vi "2_VisualizeModulePositioning2_Nolan.vi"(0 "Placement Monitor":T1(plugin-control)=refnum, 1 "Calibrated positions of fiducials [mm]":dbl[][](array[numeric])=[[-658.867386146, 115.937184375, -18.342965965], [-563.38738772, 115.95451918, -18.342965965], [-563.369748267, 18.796520782, -18.342965965], [-658.849746693, 18.779185977, -18.342965965], [-560.867387761, 115.954976697, -18.342965965], [-465.387389335, 115.972311502, -18.342965965], [-465.369749882, 18.814313103, -18.342965965], [-560.849748308, 18.796978298, -18.342965965], [-462.867389377, 115.972769019, -18.342965965], [-367.38739095, 115.990103824, -18.342965965], [-367.369751497, 18.832105425, -18.342965965], [-462.849749923, 18.81477062, -18.342965965], [-364.867390992, 115.990561341, -18.342965965], [-269.387392565, 116.007896146, -18.342965965], [-269.369753112, 18.849897747, -18.342965965], [-364.849751539, 18.832562942, -18.342965965], [-266.867392607, 116.008353663, -18.342965965], [-171.38739418, 116.025688468, -18.342965965], [-171.369754727, 18.867690069, -18.342965965], [-266.849753154, 18.850355264, -18.342965965], [-168.867394222, 116.026145985, -18.342965965], [-73.387395796, 116.04348079, -18.342965965], [-73.369756342, 18.885482391, -18.342965965], [-168.849754769, 18.868147586, -18.342965965], [-70.867395837, 116.043938306, -18.342965965], [24.612602589, 116.061273111, -18.342965965], [24.630242042, 18.903274713, -18.342965965], [-70.849756384, 18.885939908, -18.342965965], [27.132602548, 116.061730628, -18.342965965], [122.612600974, 116.079065433, -18.342965965], [122.630240427, 18.921067035, -18.342965965], [27.150242001, 18.90373223, -18.342965965], [125.132600933, 116.07952295, -18.342965965], [220.612599359, 116.096857755, -18.342965965], [220.630238812, 18.938859356, -18.342965965], [125.150240386, 18.921524551, -18.342965965], [223.132599318, 116.097315272, -18.342965965], [318.612597744, 116.114650077, -18.342965965], [318.630237197, 18.956651678, -18.342965965], [223.150238771, 18.939316873, -18.342965965], [321.132597702, 116.115107594, -18.342965965], [416.612596129, 116.132442399, -18.342965965], [416.630235582, 18.974444, -18.342965965], [321.150237156, 18.957109195, -18.342965965], [419.132596087, 116.132899916, -18.342965965], [514.612594514, 116.150234721, -18.342965965], [514.630233967, 18.992236322, -18.342965965], [419.15023554, 18.974901517, -18.342965965], [517.132594472, 116.150692238, -18.342965965], [612.612592899, 116.168027043, -18.342965965], [612.630232352, 19.010028644, -18.342965965], [517.150233925, 18.992693839, -18.342965965]], 2 "XYZ .NET Refnum in":refnum<k24>, 3 "Axis Speeds":T10={"X [mm/s]"=25.0, "Y [mm/s]"=25.0, "Z [mm/s]"=25.0}, 4 "Module fiducial marker":T7=enum."Mark C", 5 "N modules":i32=13, 6 "Sensor Pattern":T8(ring)=enum."ATLAS12", 7 "error in (no error)":errorcluster, 8 "Templates path":path=path "C:/Users/Aerotech/Documents/BNL_ThermomechanicalStave", 9 "Calibration [um/pix]":dbl=1.55, 10 "Current Build Phase":refnum<vi>, 11 "Temperature":refnum<vi>, 12 "Module #":refnum<vi>, 13 "Placement tolerance [um]":dbl=25.0, 14 "Tape Type":T5=enum."Axial (Sutcliffe NP49-01-100 01-Mar-16)", 16 "Module Report":refnum<vi>, 17 "Base notes":string, 18 "Reports path":path=path "C:/Users/Aerotech/cernbox/BNL/Stave Assembly Records/2017-05-15/ModulePlacement") -> (19 "Recalibrated??":bool, 22 "XYZ .NET Refnum out":refnum<k24>, 27 "error out":errorcluster)   [LabVIEW 2016] (continued)
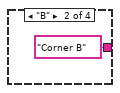
[diagram p4: hidden frame]
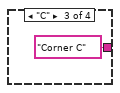
[diagram p5: hidden frame]
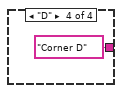
[diagram p6: hidden frame]
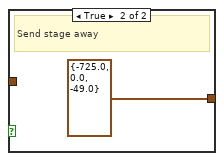
[diagram p7: hidden frame]
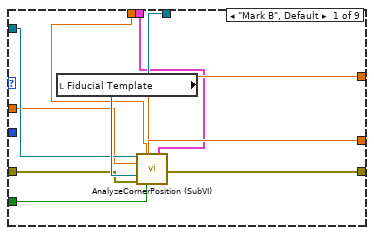
[diagram p8: hidden frame]
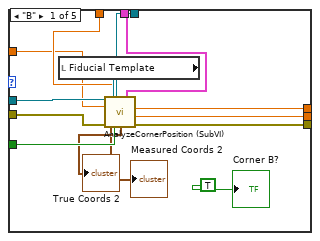
[diagram p9: hidden frame]
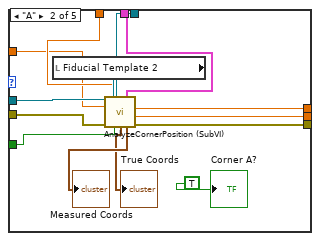
[diagram p10: hidden frame]
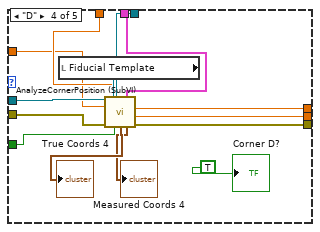
[diagram p11: hidden frame]
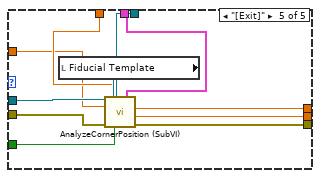
[diagram p12: hidden frame]
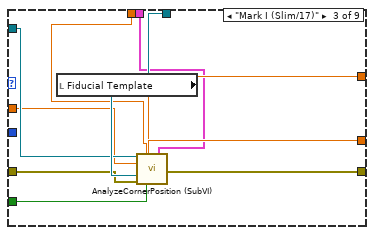
[diagram p13: hidden frame]
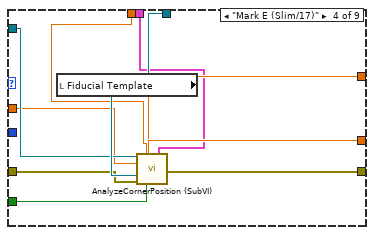
[diagram p14: hidden frame]
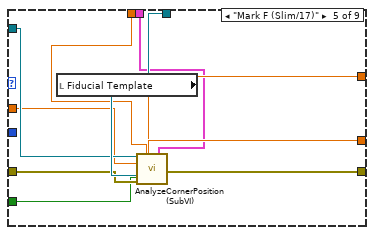
[diagram p15: hidden frame]
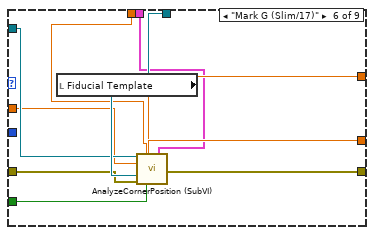
[diagram p16: hidden frame]
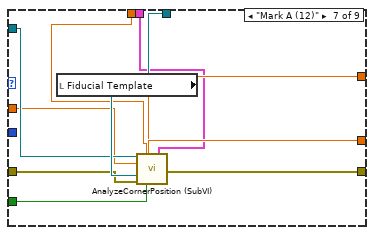
[diagram p17: hidden frame]
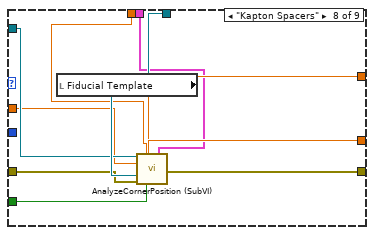
[diagram p18: hidden frame]
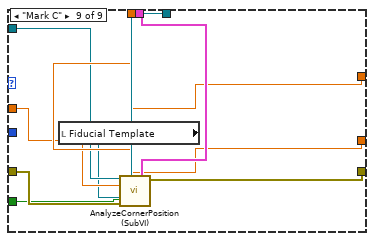
[diagram p19: hidden frame]
                                "Corner B?" <- TRUE
                              }
                              frame "A" {
                                n57 = local read "Fiducial Template 2"() -> (w249:T1)
                                n58 = call "AnalyzeCornerPosition (SubVI).vi"("Refnum in"=w244, "Placement tolerance [um]"=w242, "Calibration [um/pix]"=w240, "Fiducial Template"=w249, "error in (no error)"=w248, "Center-only search?"=w239) -> ("Offset interpreter"=w241:T3, "Refnum out"=w243:T1, "X offset [um]"=w245:sgl, "Y offset [um]"=w246:sgl, "True Coords"=→"True Coords":cluster{"X coordinate":dbl, "Y coordinate":dbl}, "Measured Coords"=→"Measured Coords":cluster{"x":sgl, "y":sgl}, "error out"=w247:errorcluster)  [unwired: 3 in]
                                "Corner A?" <- TRUE
                              }
                              frame "C" {
                                n59 = local read "Fiducial Template 2"() -> (w263:T1)
                                n60 = call "AnalyzeCornerPosition (SubVI).vi"("Refnum in"=w258, "Placement tolerance [um]"=w256, "Calibration [um/pix]"=w254, "Fiducial Template"=w263, "error in (no error)"=w262, "Center-only search?"=w253) -> ("Offset interpreter"=w255:T3, "Refnum out"=w257:T1, "X offset [um]"=w259:sgl, "Y offset [um]"=w260:sgl, "True Coords"=→"True Coords 3":cluster{"X coordinate":dbl, "Y coordinate":dbl}, "Measured Coords"=→"Measured Coords 3":cluster{"x":sgl, "y":sgl}, "error out"=w261:errorcluster)  [unwired: 3 in]
                                "Corner C?" <- TRUE
                              }
                              frame "D" {
                                n61 = local read "Fiducial Template"() -> (w277:T1)
                                n62 = call "AnalyzeCornerPosition (SubVI).vi"("Refnum in"=w272, "Placement tolerance [um]"=w270, "Calibration [um/pix]"=w268, "Fiducial Template"=w277, "error in (no error)"=w276, "Center-only search?"=w267) -> ("Offset interpreter"=w269:T3, "Refnum out"=w271:T1, "X offset [um]"=w273:sgl, "Y offset [um]"=w274:sgl, "True Coords"=→"True Coords 4":cluster{"X coordinate":dbl, "Y coordinate":dbl}, "Measured Coords"=→"Measured Coords 4":cluster{"x":sgl, "y":sgl}, "error out"=w275:errorcluster)  [unwired: 3 in]
                                "Corner D?" <- TRUE
                              }
                              frame "[Exit]" {
                                n63 = local read "Fiducial Template"() -> (w288:T1)
                                n64 = call "AnalyzeCornerPosition (SubVI).vi"("Refnum in"=w283, "Placement tolerance [um]"=w281, "Calibration [um/pix]"=w279, "Fiducial Template"=w288, "error in (no error)"=w287, "Center-only search?"=w278) -> ("Offset interpreter"=w280:T3, "Refnum out"=w282:T1, "X offset [um]"=w284:sgl, "Y offset [um]"=w285:sgl, "error out"=w286:errorcluster)  [unwired: 3 in, 2 out]
                              }
                            }
                          }
                          frame "Mark I (Slim/17)" {
                            n65 = local read "Fiducial Template"() -> (w299:T1)
                            n66 = call "AnalyzeCornerPosition (SubVI).vi"("Refnum in"=w294, "Placement tolerance [um]"=w292, "Calibration [um/pix]"=w290, "Fiducial Template"=w299, "error in (no error)"=w298, "Center-only search?"=w289) -> ("Offset interpreter"=w291:T3, "Refnum out"=w293:T1, "X offset [um]"=w295:sgl, "Y offset [um]"=w296:sgl, "error out"=w297:errorcluster)  [unwired: 3 in, 2 out]
                          }
                          frame "Mark E (Slim/17)" {
                            n67 = local read "Fiducial Template"() -> (w310:T1)
                            n68 = call "AnalyzeCornerPosition (SubVI).vi"("Refnum in"=w305, "Placement tolerance [um]"=w303, "Calibration [um/pix]"=w301, "Fiducial Template"=w310, "error in (no error)"=w309, "Center-only search?"=w300) -> ("Offset interpreter"=w302:T3, "Refnum out"=w304:T1, "X offset [um]"=w306:sgl, "Y offset [um]"=w307:sgl, "error out"=w308:errorcluster)  [unwired: 3 in, 2 out]
                          }
                          frame "Mark F (Slim/17)" {
                            n69 = local read "Fiducial Template"() -> (w321:T1)
                            n70 = call "AnalyzeCornerPosition (SubVI).vi"("Refnum in"=w316, "Placement tolerance [um]"=w314, "Calibration [um/pix]"=w312, "Fiducial Template"=w321, "error in (no error)"=w320, "Center-only search?"=w311) -> ("Offset interpreter"=w313:T3, "Refnum out"=w315:T1, "X offset [um]"=w317:sgl, "Y offset [um]"=w318:sgl, "error out"=w319:errorcluster)  [unwired: 3 in, 2 out]
                          }
                          frame "Mark G (Slim/17)" {
                            n71 = local read "Fiducial Template"() -> (w332:T1)
                            n72 = call "AnalyzeCornerPosition (SubVI).vi"("Refnum in"=w327, "Placement tolerance [um]"=w325, "Calibration [um/pix]"=w323, "Fiducial Template"=w332, "error in (no error)"=w331, "Center-only search?"=w322) -> ("Offset interpreter"=w324:T3, "Refnum out"=w326:T1, "X offset [um]"=w328:sgl, "Y offset [um]"=w329:sgl, "error out"=w330:errorcluster)  [unwired: 3 in, 2 out]
                          }
                          frame "Mark A (12)" {
                            n73 = local read "Fiducial Template"() -> (w343:T1)
                            n74 = call "AnalyzeCornerPosition (SubVI).vi"("Refnum in"=w338, "Placement tolerance [um]"=w336, "Calibration [um/pix]"=w334, "Fiducial Template"=w343, "error in (no error)"=w342, "Center-only search?"=w333) -> ("Offset interpreter"=w335:T3, "Refnum out"=w337:T1, "X offset [um]"=w339:sgl, "Y offset [um]"=w340:sgl, "error out"=w341:errorcluster)  [unwired: 3 in, 2 out]
                          }
                          frame "Kapton Spacers" {
                            n75 = local read "Fiducial Template"() -> (w354:T1)
                            n76 = call "AnalyzeCornerPosition (SubVI).vi"("Refnum in"=w349, "Placement tolerance [um]"=w347, "Calibration [um/pix]"=w345, "Fiducial Template"=w354, "error in (no error)"=w353, "Center-only search?"=w344) -> ("Offset interpreter"=w346:T3, "Refnum out"=w348:T1, "X offset [um]"=w350:sgl, "Y offset [um]"=w351:sgl, "error out"=w352:errorcluster)  [unwired: 3 in, 2 out]
                          }
                          frame "Mark C" {
                            n77 = local read "Fiducial Template"() -> (w355:T1)
                            n78 = call "AnalyzeCornerPosition (SubVI).vi"("Refnum in"=w362, "Placement tolerance [um]"=w363, "Calibration [um/pix]"=w361, "Fiducial Template"=w355, "error in (no error)"=w357, "Center-only search?"=w356) -> ("Offset interpreter"=w360:T3, "Refnum out"=w364:T1, "X offset [um]"=w359:sgl, "Y offset [um]"=w358:sgl, "error out"=w365:errorcluster)  [unwired: 3 in, 2 out]
                          }
                        }
                        "X offset [um]" <- w192
                        "Y offset [um]" <- w191
                        "Offset interpreter" <- w193
                        n79 = local write "Placement Monitor"(w197) -> ()
                      }
                    }
                    frame True {
                    }
                  }
                }
                frame #3 {
                  # "Update the module progress report"
                  n80 = local read "Module Progress Report"() -> (w371:T11)
                  n81 = local read "Module Report"() -> (w374:refnum<vi>)
                  n82 = Replace Array Subset(array=w371, new element="User Report: Current Module", index=w370) -> (w372:T11)
                  n83 = property class="Ctl"(reference=w374, error in=w368, "Value"=w372) -> (error out=w367:errorcluster)  [unwired: 1 out]
                  n84 = local write "Module Progress Report"(w372) -> ()
                }
              }
            }
            frame True {
              # "Exit module alignment to do a survey or apply glue"
              n85 = disable-structure shown="Enabled" {
                disable-tunnel: w379 -> [w386 _]
                disable-tunnel: w378 -> [w382 w392]
                disable-tunnel: [w381 w391] -> w377
                frame Disabled {
                  n86 = local read "User Report: Current Module"() -> (w390:T4)
                  n87 = local read "Module Progress Report"() -> (w387:T11)
                  n88 = local read "Module Report"() -> (w389:refnum<vi>)
                  n89 = Replace Array Subset(array=w387, new element=w390, index=w386) -> (w388:T11)
                  n90 = property class="Ctl"(reference=w389, error in=w382, "Value"=w388) -> (error out=w383:errorcluster)  [unwired: 1 out]
                  n91 = local write "Module Progress Report"(w388) -> ()
                  n92 = property on="Module corner loop stop" class="Bool"(error in=w383, "BoolText.Text"="Waiting..." ("Boolean Text.Text"), "DisabledEnum"=T12."Disabled and Grayed Out" ("Disabled")) -> (error out=w381:errorcluster)  [unwired: 1 in, 1 out]
                }
                frame Enabled {
                  n93 = property on="Module corner loop stop" class="Bool"(error in=w392, "BoolText.Text"="Waiting..." ("Boolean Text.Text"), "DisabledEnum"=T12."Disabled and Grayed Out" ("Disabled")) -> (error out=w391:errorcluster)  [unwired: 1 in, 1 out]
                }
              }
              n94 = local read "Send XYZ stage beyond EOS"() -> (w375:bool)
              n95 = case "Select destination coordinates" shown="False" w375 {
                tunnel: w377 -> [w395 w400]
                tunnel: [w395 w399] -> w376
                frame False {
                  # "Go to corner"
                }
                frame True {
                  # "Send stage away"
                  n96 = local read "XYZ .NET Refnum in"() -> (w397:refnum<k24>)
                  n97 = local read "Axis Speeds"() -> (w401:T10)
                  n98 = call "Go2XYZ (SubVI).vi"(".NET Refnum in"=w397, "Go to Coordinates"=cluster{"X":dbl, "Y":dbl, "Z":dbl} {"X"=-725.0, "Y"=0.0, "Z"=-49.0}, "Axis Speeds"=w401, "error in (no error)"=w400) -> (".NET Refnum out"=w398:refnum<k24>, "Final Position"=w396:T14, "error out"=w399:errorcluster)  [unwired: 7 in, 2 out]
                  n99 = local write "XYZ .NET Refnum out"(w398) -> ()
                  n100 = local write "Current Stage Position"(w396) -> ()
                }
              }
            }
          }
          "Current task:" <- "Aligning modules..." ("Prgm dialogue")
        }
        n101 = local read "Exit to survey or glue"() -> (w86:bool)
        n102 = local read "Measured Coords 2"() -> (w77:cluster{"X coordinate":sgl, "Y coordinate":sgl})
        n103 = local read "Measured Coords 3"() -> (w78:cluster{"X coordinate":sgl, "Y coordinate":sgl})
        n104 = local read "Measured Coords 4"() -> (w79:cluster{"X coordinate":sgl, "Y coordinate":sgl})
        n105 = local read "Corner D?"() -> (w69:bool)
        n106 = local read "Corner A?"() -> (w71:bool)
        n107 = local read "Corner C?"() -> (w70:bool)
        n108 = local read "Corner B?"() -> (w72:bool)
        n109 = local read "Measured Coords"() -> (w76:cluster{"X coordinate":sgl, "Y coordinate":sgl})
        n110 = local read "True Coords 2"() -> (w81:cluster{"X coordinate":dbl, "Y coordinate":dbl})
        n111 = local read "True Coords 3"() -> (w82:cluster{"X coordinate":dbl, "Y coordinate":dbl})
        n112 = local read "True Coords 4"() -> (w83:cluster{"X coordinate":dbl, "Y coordinate":dbl})
        n113 = local read "True Coords"() -> (w80:cluster{"X coordinate":dbl, "Y coordinate":dbl})
        n114 = And(x=w71, y=w72) -> (x .and. y?=w74:bool)
        n115 = And(x=w70, y=w69) -> (x .and. y?=w73:bool)
        n116 = And(x=w74, y=w73) -> (x .and. y?=w75:bool)
        n117 = Bundle("Measured Coords"=w76, "Measured Coords 2"=w77, "Measured Coords 3"=w78, "Measured Coords 4"=w79) -> (w85:T15)  [unwired: 1 in]
        n118 = Bundle("True Coords"=w80, "True Coords 2"=w81, "True Coords 3"=w82, "True Coords 4"=w83) -> (w84:T16)  [unwired: 1 in]
        n119 = case shown="True" w75 {
          tunnel: w85 -> [_ w93]
          tunnel: w84 -> [_ w92]
          frame False {
          }
          frame True {
            n120 = call "KnobTurns.vi"("Expected Corner Positions"=w92, "Measured Corner Positions"=w93) -> ("Y/Angle Knob Turns"=→"Y Knob Turns":dbl, "X/Pos Knob Turns"=→"X Knob Turns":cluster{"X":dbl, "Y":dbl})  [unwired: 1 in]
          }
        }
      }
      frame #1 {
        n121 = case shown="False" w403 {
          tunnel: [T13."Right Button" ("Which Button?") w415] -> w406
          frame False {
          }
          frame True {
            n122 = local read "Assembly step"() -> (w411:string)
            n123 = local read "Module # str"() -> (w414:string)
            n124 = local write "Exit to survey or glue"(FALSE ("Exit to survey or glue")) -> ()
            n125 = Concatenate Strings("Would you like to survey or glue " ("message"), w414, "? Survey results will be labeled \"" ("string"), w411, ".\"" ("string")) -> (w409:string)
            n126 = call <vilib>:"Three Button Dialog.vi"("Right Button Text (\"Cancel\")"="Cancel" ("Right Button Text (\"Cancel\")"), "Center Button Text (\"No\")"="Apply glue" ("Center Button Text (\"No\")"), "Left Button Text (\"Yes\")"="Survey" ("Left Button Text (\"Yes\")"), "message"=w409) -> ("Which Button?"=w415:T13)  [unwired: 7 in]
          }
        }
      }
      frame #2 {
        n127 = case shown="\"Left Button\"" w422 {
          tunnel: w421 -> [w444 w666 _]
          tunnel: [w432 w668 w689] -> w420
          tunnel: w419 -> [w428 w663 w689]
          frame "Left Button" {
            # "Do a survey"
            n128 = local read "Work on Module #..."() -> (w426:i32)
            n129 = local read "Module # str"() -> (w424:string)
            n130 = local read "Module Progress Report"() -> (w437:T11)
            n131 = Concatenate Strings("Surveying " ("Prgm dialogue"), w424) -> (w423:string)
            n132 = Number To Decimal String(number=w426) -> (decimal integer string=w445:string)  [unwired: 1 in]
            n133 = Decrement(x=w426) -> (x-1=w429:i32)
            n134 = local write "Current task:"(w423) -> ()
            n135 = call "RecursiveDirectoryStructureGenerator (SubVI).vi"("error in (no error)"=w428, "Folder index"=w426, "Host directory"="Reports path") -> ("error out"=w427:errorcluster, "Nth subfolder in host directory"=w431:path)  [unwired: 7 in]
            n136 = Index Array(array=w437, index=w429) -> (element=w435:T4)
            n137 = Concatenate Strings("Module_" ("string"), w445) -> (w433:string)
            n138 = Index Array(array=w444, index (row)=w429) -> (element=w446:cluster{"X":dbl, "Y":dbl, "Z":dbl}[])  [unwired: 1 in]
            n139 = for "Survey and save a corner of the module" {
              tunnel: w431 -> [w472]
              tunnel: [w485] -> w443 mode=indexing
              tunnel: w446 -> [w457] mode=indexing
              tunnel: string[] ["A", "B", "C", "D"] -> [w453] mode=indexing
              tunnel: w435 -> [w479]
              tunnel: w433 -> [w460]
              tunnel: w427 -> [w459]
              w462 = "_" ("string")
              n140 = local read "Placement tolerance [um]"() -> (w483:dbl)
              n141 = local read "Module fiducial marker"() -> (w455:T7)
              n142 = local read "Manual Z?"() -> (w456:bool)
              n143 = local read "Calibration [um/pix]"() -> (w482:dbl)
              n144 = local read "XYZ .NET Refnum in"() -> (w488:refnum<k24>)
              n145 = local read "Placement Monitor"() -> (w484:T1)
              n146 = local read "Axis Speeds"() -> (w481:T10)
              n147 = Unbundle By Name(w479) -> ("ID"=w478:string)
              n148 = local read "Assembly step"() -> (w461:string)
              n149 = case shown="True" w456 {
                tunnel: w457 -> [w632 w637]
                tunnel: [w632 w633] -> w458
                frame False {
                }
                frame True {
                  n150 = local read "Manual Z [mm]"() -> (w634:dbl)
                  n151 = Unbundle By Name(w637) -> ("X"=w636:dbl, "Y"=w635:dbl)
                  n152 = Bundle("X"=w636, "Y"=w635, "Manual Z [mm]"=w634) -> (w633:cluster{"X":dbl, "Y":dbl, "Manual Z [mm]":dbl})  [unwired: 1 in]
                }
              }
              n153 = Concatenate Strings(w460, ".txt" ("string")) -> (w474:string)
              n154 = Equal?(x=w453, y="A") -> (x = y?=w450:bool)
              n155 = Equal?(x=w453, y="C") -> (x = y?=w451:bool)
              n156 = Build Path(base path=w472, name or relative path=w474) -> (appended path=w473:path)
              n157 = Concatenate Strings("Corner" ("string"), w453) -> (w470:string)
              n158 = Or(x=w450, y=w451) -> (x .or. y?=w449:bool)
              n159 = case shown="\"Mark B\"" w455 {
                tunnel: w488 -> [w501 w514 w527 w566 w579 w592 w605 w618 w631]
                tunnel: [w499 w512 w526 w564 w577 w590 w603 w616 w629] -> w486
                tunnel: w484 -> [w498 w511 w525 w563 w576 w589 w602 w615 w628]
                tunnel: w483 -> [w497 w510 w524 w562 w575 w588 w601 w614 w627]
                tunnel: w482 -> [w496 w509 w523 w561 w574 w587 w600 w613 w626]
                tunnel: w481 -> [w495 w508 w522 w560 w573 w586 w599 w612 w625]
                tunnel: [w494 w507 w521 w559 w572 w585 w598 w611 w624] -> w467
                tunnel: [w493 w506 w520 w558 w571 w584 w597 w610 w623] -> w465
                tunnel: [w492 w505 w519 w557 w570 w583 w596 w609 w622] -> w464
                tunnel: [w491 w504 w518 w556 w569 w582 w595 w608 w621] -> w463
                tunnel: w459 -> [w490 w503 w517 w555 w568 w581 w594 w607 w620]
                tunnel: w458 -> [w489 w502 w516 w554 w567 w580 w593 w606 w619]
                tunnel: w449 -> [_ _ w515 _ _ _ _ _ _]
                frame "Mark C", Default {
                  n160 = local read "Fiducial Template"() -> (w500:T1)
                  n161 = call "CollectCorner (SubVI).vi"("XYZ .NET Refnum in"=w501, "Calibration [um/pix]"=w496, "Placement tolerance [um]"=w497, "Placement Monitor"=w498, "Fiducial Template"=w500, "error in (no error)"=w490, "Axis Speeds"=w495, "Corner Coordinates"=w489) -> ("XYZ .NET Refnum out"=w491:refnum<k24>, "Placement Monitor out"=w492:T1, "Corner surveyed position"=w494:dbl[], "XYZ Stage Final Position"=w493:T14, "error out"=w499:errorcluster)  [unwired: 3 in]
                }
                frame "Mark B" {
                  n162 = local read "Fiducial Template"() -> (w513:T1)
                  n163 = call "CollectCorner (SubVI).vi"("XYZ .NET Refnum in"=w514, "Calibration [um/pix]"=w509, "Placement tolerance [um]"=w510, "Placement Monitor"=w511, "Fiducial Template"=w513, "error in (no error)"=w503, "Axis Speeds"=w508, "Corner Coordinates"=w502) -> ("XYZ .NET Refnum out"=w504:refnum<k24>, "Placement Monitor out"=w505:T1, "Corner surveyed position"=w507:dbl[], "XYZ Stage Final Position"=w506:T14, "error out"=w512:errorcluster)  [unwired: 3 in]
                }
                frame "Bias Ring Corner" {
                  n164 = case shown="True" w515 {
                    tunnel: w527 -> [w540 w553]
                    tunnel: [w538 w551] -> w526
                    tunnel: w525 -> [w537 w550]
                    tunnel: w524 -> [w536 w549]
                    tunnel: w523 -> [w535 w548]
                    tunnel: w522 -> [w534 w547]
                    tunnel: [w533 w546] -> w521
                    tunnel: [w532 w545] -> w520
                    tunnel: [w531 w544] -> w519
                    tunnel: [w530 w543] -> w518
                    tunnel: w517 -> [w529 w542]
                    tunnel: w516 -> [w528 w541]
                    frame True {
                      n165 = local read "Fiducial Template 2"() -> (w539:T1)
                      n166 = call "CollectCorner (SubVI).vi"("XYZ .NET Refnum in"=w540, "Calibration [um/pix]"=w535, "Placement tolerance [um]"=w536, "Placement Monitor"=w537, "Fiducial Template"=w539, "error in (no error)"=w529, "Axis Speeds"=w534, "Corner Coordinates"=w528) -> ("XYZ .NET Refnum out"=w530:refnum<k24>, "Placement Monitor out"=w531:T1, "Corner surveyed position"=w533:dbl[], "XYZ Stage Final Position"=w532:T14, "error out"=w538:errorcluster)  [unwired: 3 in]
                    }
                    frame False {
                      n167 = local read "Fiducial Template"() -> (w552:T1)
                      n168 = call "CollectCorner (SubVI).vi"("XYZ .NET Refnum in"=w553, "Calibration [um/pix]"=w548, "Placement tolerance [um]"=w549, "Placement Monitor"=w550, "Fiducial Template"=w552, "error in (no error)"=w542, "Axis Speeds"=w547, "Corner Coordinates"=w541) -> ("XYZ .NET Refnum out"=w543:refnum<k24>, "Placement Monitor out"=w544:T1, "Corner surveyed position"=w546:dbl[], "XYZ Stage Final Position"=w545:T14, "error out"=w551:errorcluster)  [unwired: 3 in]
                    }
                  }
                }
                frame "Mark I (Slim/17)" {
                  n169 = local read "Fiducial Template"() -> (w565:T1)
                  n170 = call "CollectCorner (SubVI).vi"("XYZ .NET Refnum in"=w566, "Calibration [um/pix]"=w561, "Placement tolerance [um]"=w562, "Placement Monitor"=w563, "Fiducial Template"=w565, "error in (no error)"=w555, "Axis Speeds"=w560, "Corner Coordinates"=w554) -> ("XYZ .NET Refnum out"=w556:refnum<k24>, "Placement Monitor out"=w557:T1, "Corner surveyed position"=w559:dbl[], "XYZ Stage Final Position"=w558:T14, "error out"=w564:errorcluster)  [unwired: 3 in]
                }
                frame "Mark E (Slim/17)" {
                  n171 = local read "Fiducial Template"() -> (w578:T1)
                  n172 = call "CollectCorner (SubVI).vi"("XYZ .NET Refnum in"=w579, "Calibration [um/pix]"=w574, "Placement tolerance [um]"=w575, "Placement Monitor"=w576, "Fiducial Template"=w578, "error in (no error)"=w568, "Axis Speeds"=w573, "Corner Coordinates"=w567) -> ("XYZ .NET Refnum out"=w569:refnum<k24>, "Placement Monitor out"=w570:T1, "Corner surveyed position"=w572:dbl[], "XYZ Stage Final Position"=w571:T14, "error out"=w577:errorcluster)  [unwired: 3 in]
                }
                frame "Mark F (Slim/17)" {
                  n173 = local read "Fiducial Template"() -> (w591:T1)
                  n174 = call "CollectCorner (SubVI).vi"("XYZ .NET Refnum in"=w592, "Calibration [um/pix]"=w587, "Placement tolerance [um]"=w588, "Placement Monitor"=w589, "Fiducial Template"=w591, "error in (no error)"=w581, "Axis Speeds"=w586, "Corner Coordinates"=w580) -> ("XYZ .NET Refnum out"=w582:refnum<k24>, "Placement Monitor out"=w583:T1, "Corner surveyed position"=w585:dbl[], "XYZ Stage Final Position"=w584:T14, "error out"=w590:errorcluster)  [unwired: 3 in]
                }
                frame "Mark G (Slim/17)" {
                  n175 = local read "Fiducial Template"() -> (w604:T1)
                  n176 = call "CollectCorner (SubVI).vi"("XYZ .NET Refnum in"=w605, "Calibration [um/pix]"=w600, "Placement tolerance [um]"=w601, "Placement Monitor"=w602, "Fiducial Template"=w604, "error in (no error)"=w594, "Axis Speeds"=w599, "Corner Coordinates"=w593) -> ("XYZ .NET Refnum out"=w595:refnum<k24>, "Placement Monitor out"=w596:T1, "Corner surveyed position"=w598:dbl[], "XYZ Stage Final Position"=w597:T14, "error out"=w603:errorcluster)  [unwired: 3 in]
                }
                frame "Mark A (12)" {
                  n177 = local read "Fiducial Template"() -> (w617:T1)
                  n178 = call "CollectCorner (SubVI).vi"("XYZ .NET Refnum in"=w618, "Calibration [um/pix]"=w613, "Placement tolerance [um]"=w614, "Placement Monitor"=w615, "Fiducial Template"=w617, "error in (no error)"=w607, "Axis Speeds"=w612, "Corner Coordinates"=w606) -> ("XYZ .NET Refnum out"=w608:refnum<k24>, "Placement Monitor out"=w609:T1, "Corner surveyed position"=w611:dbl[], "XYZ Stage Final Position"=w610:T14, "error out"=w616:errorcluster)  [unwired: 3 in]
                }
                frame "Kapton Spacers" {
                  n179 = local read "Fiducial Template"() -> (w630:T1)
                  n180 = call "CollectCorner (SubVI).vi"("XYZ .NET Refnum in"=w631, "Calibration [um/pix]"=w626, "Placement tolerance [um]"=w627, "Placement Monitor"=w628, "Fiducial Template"=w630, "error in (no error)"=w620, "Axis Speeds"=w625, "Corner Coordinates"=w619) -> ("XYZ .NET Refnum out"=w621:refnum<k24>, "Placement Monitor out"=w622:T1, "Corner surveyed position"=w624:dbl[], "XYZ Stage Final Position"=w623:T14, "error out"=w629:errorcluster)  [unwired: 3 in]
                }
              }
              n181 = local read "Mark string"() -> (w477:string)
              n182 = Concatenate Strings(w460, w462, w461, w462, w470, ".png" ("string")) -> (w469:string)
              n183 = local write "Placement Monitor"(w464) -> ()
              n184 = local write "Current Stage Position"(w465) -> ()
              n185 = local write "XYZ .NET Refnum out"(w463) -> ()
              n186 = Bundle("ID"=w478, "Mark string"=w477, "Assembly step"=w461, "User notes"="User notes", w470, "Corner surveyed position"=w467) -> (w466:T17)  [unwired: 1 in]
              n187 = Build Path(base path=w472, name or relative path=w469) -> (appended path=w468:path)
              n188 = property class="Slide (strict)"(reference="Temperature") -> ("Value"=w447:dbl)  [unwired: 1 in, 2 out]
              n189 = call "SaveCorner (SubVI).vi"("Module record filename"=w473, "Temperature"=w447, "Write to file"=TRUE, "Data strings"=w466, "Module corner image filename"=w468, "Image of corner"=w464, "error in (no error)"=w486) -> ("error out"=w485:errorcluster)  [unwired: 8 in]
            }
            n190 = local read "User Report: Current Module"() -> (w442:T4)
            n191 = local read "Module Progress Report"() -> (w439:T11)
            n192 = Replace Array Subset(array=w439, new element=w442, index=w429) -> (w440:T11)
            n193 = local write "Module Progress Report"(w440) -> ()
            n194 = local read "Module Report"() -> (w441:refnum<vi>)
            n195 = Merge Errors(w443) -> (w438:errorcluster)
            n196 = property class="Ctl"(reference=w441, error in=w438, "Value"=w440) -> (error out=w432:errorcluster)  [unwired: 1 out]
          }
          frame "Center Button" {
            # "Apply glue lives here"
            # "Apply Glue"
            n197 = local read "Module # str"() -> (w643:string)
            n198 = local read "Work on Module #..."() -> (w649:i32)
            n199 = Concatenate Strings("Applying glue for " ("Prgm dialogue"), w643) -> (w642:string)
            n200 = local write "Current task:"(w642) -> ()
            n201 = Decrement(x=w649) -> (x-1=w667:i32)
            n202 = Index Array(array=w666, index (row)=w667) -> (element=w665:cluster{"X":dbl, "Y":dbl, "Z":dbl}[])  [unwired: 1 in]
            n203 = for {
              tunnel: w665 -> [w688] mode=indexing
              tunnel: [w687] -> w664 mode=indexing
              n204 = Cluster To Array(cluster=w688) -> (array=w687:dbl[])
            }
            n205 = local read "Reports path"() -> (w650:path)
            n206 = call "GetModuleCentre (SubVI).vi"("error in (no error)"=w663, "4x3 Array of Fiducial Coordinates"=w664) -> ("error out"=w648:errorcluster, "y, centre"=w659:dbl, "x, centre"=w662:dbl)  [unwired: 1 in]
            n207 = call "RecursiveDirectoryStructureGenerator (SubVI).vi"("error in (no error)"=w648, "Folder index"=w649, "Host directory"=w650) -> ("error out"=w647:errorcluster, "Nth subfolder in host directory"=w639:path)  [unwired: 7 in]
            n208 = local read "Templates path"() -> (w645:path)
            n209 = Add(x=w662, y=-45.0) -> (x+y=w657:dbl)
            n210 = local read "Calibration [um/pix]"() -> (w658:dbl)
            n211 = local read "XYZ .NET Refnum in"() -> (w653:refnum<k24>)
            n212 = local read "Placement Monitor"() -> (w651:T1)
            n213 = Add(x=w659, y=45.0) -> (x+y=w656:dbl)
            n214 = Bundle(w657, w656, "y"=-49.0) -> (w654:cluster{dbl, dbl, "y":dbl})  [unwired: 1 in]
            n215 = Build Path(base path=w645, name or relative path="Utils\\ConfigurationFiles_and_Templates\\1_ModulePlacement") -> (appended path=w644:path)
            n216 = case shown="False" "Dots (T) or Lines (F)" {
              tunnel: [w670 w686] -> w668
              tunnel: w658 -> [w676 w685]
              tunnel: w654 -> [w674 w684]
              tunnel: w653 -> [w673 w683]
              tunnel: [w672 w682] -> w652
              tunnel: w651 -> [w671 w681]
              tunnel: w647 -> [w675 w680]
              tunnel: w644 -> [w669 w679]
              tunnel: "Tape Type" -> [_ w678]
              tunnel: w639 -> [_ w677]
              frame False {
                n217 = call "Alyssa_GlueFatLines.vi"("Image Feed"=w671, "Template Path"=w669, "error in"=w675, "um/pix resolution"=w676, "Module corner coordinates"=w674, "XYZ Stage Control"=w673) -> ("error out"=w670:errorcluster, "XYZ .NET Refnum out"=w672:refnum<k24>)  [unwired: 4 in]
              }
              frame True {
                n218 = call "GlueSingleModule(SubVI).vi"("XYZ Stage Control"=w683, "Template Path"=w679, "Image Feed"=w681, "Module corner coordinates"=w684, "Path to save collected images"=w677, "um/pix resolution"=w685, "error in"=w680, "Tape Type"=w678) -> ("XYZ .NET Refnum out"=w682:refnum<k24>, "error out"=w686:errorcluster)  [unwired: 6 in]
              }
            }
            n219 = local write "XYZ .NET Refnum out"(w652) -> ()
          }
          frame "Right Button", Default {
            # "Do nothing -- go back to positioning modules"
            # "Do nothing (exit or return to module alignment)"
          }
        }
      }
    }
  }
  n220 = local read "Fiducial Template"() -> (w26:T1)
  n221 = call "IMAQ Dispose"("Image"=w26, "error in (no error)"=w5) -> ("error out"=w25:errorcluster)  [unwired: 4 in]
  n222 = call <vilib>:"General Error Handler.vi"("error in (no error)"=w25) -> ("error out"=→"error out":errorcluster)  [unwired: 10 in, 4 out]
  "Module Progress Report" <- T11 [] ("Module Progress Report")
